vi "CRYO_MASTER_temp.vi"() -> ()   [LabVIEW 2017] (continued)
  out "LastMeasurementConfig (336)":T10(array[cluster])=[{"LSIName"="LSi336X", "Active?"=TRUE, "LastData"=[295.892, 295.621, 295.543, 295.514], "Labels"=["T1K3-1", "T1K3-2", "T3He5", "T3He8"]}, {"LSIName"="LSi336Y", "Active?"=TRUE, "LastData"=[295.418, 295.377, 295.467, 295.916], "Labels"=["T3He6-1", "T3He6-2", "T3He7-1", "T3He7-2"]}]
  out "DataArrayConv (USB) 2":dbl[][](array[numeric])
  # "GLOBAL STATUS/CONTROL"
  # "USB6210 Analog inputs Settings"
  # "USB6218 Analog inputs Settings"
  # "USB6218 Dewar Pressure Regulation"
  # "Global Settings"
  # "LSI218 Settings"
  # "LSI336 Settings"
  # "LSI218 Settings"
  # "Graph screenshots"
  # "Configuration"
  # "Vavle Status"
  # "OPEN"
  # "CLOSED"
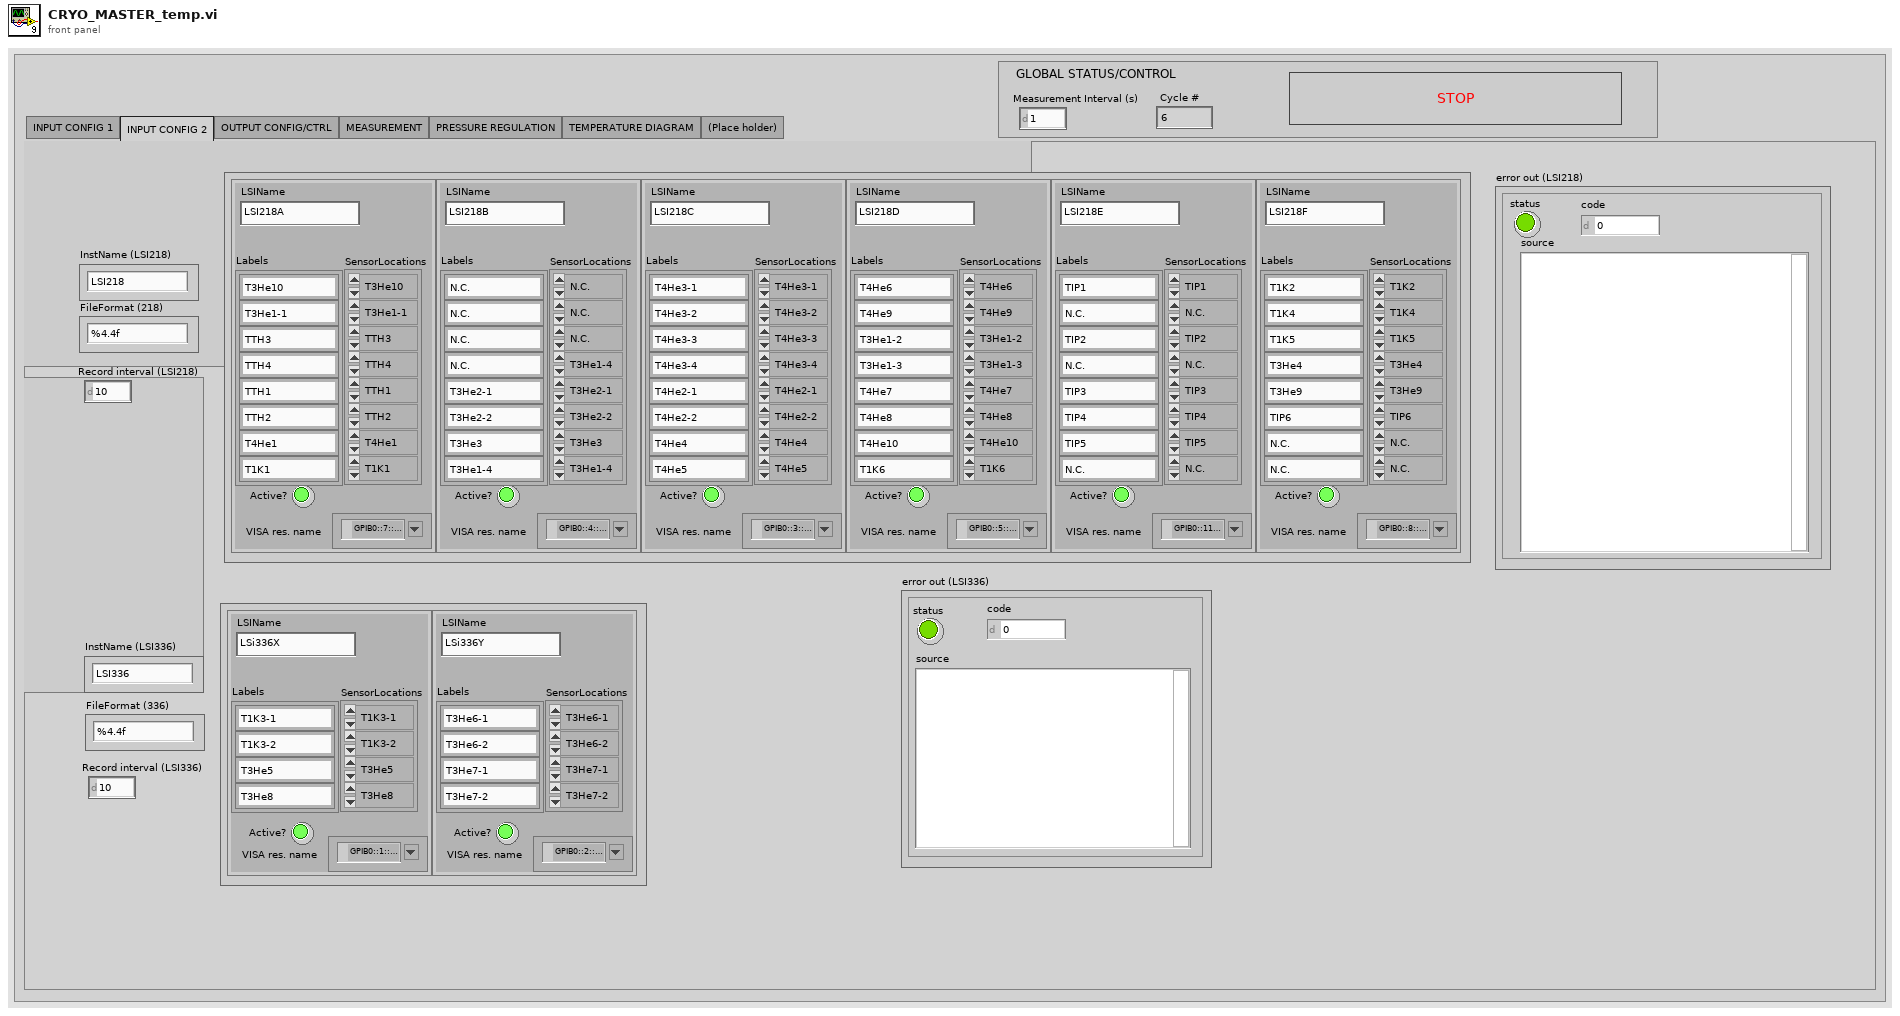
[diagram p1: front panel]
types:
  T1 = enum32{"INPUT CONFIG 1", "INPUT CONFIG 2", "OUTPUT CONFIG/CTRL", "MEASUREMENT", "PRESSURE REGULATION", "TEMPERATURE DIAGRAM", "(Place holder)"}
  T2 = cluster{"Label":string, "FileFormat":string, "Active?":bool, "Physical CH":tag, " terminal\n type":i32, "ConversionType":cluster{"Type":enum16{"Raw", "SimpleProp", "CC-10_COMBINED", "CC-10_LOG", "LeakDet_EXP", "LeakDet_Mantissa", "Baratron"}, "ConversionParameters":dbl[]}, "VoltageLimits":dbl[]}[]
  T3 = cluster{"LSIName":string, "Labels":string[], "SensorLocations":enum16{"N.C.", "T3He1-1", "T3He1-2", "T3He1-3", "T3He1-4", "T3He2-1", "T3He2-2", "T3He3", "T3He4", "T3He5", "T3He6-1", "T3He6-2", "T3He7-1", "T3He7-2", "T3He8", "T3He9", "T3He10", "T4He1", "T4He2-1", "T4He2-2", "T4He3-1", "T4He3-2", "T4He3-3", "T4He3-4", "T4He4", "T4He5", "T4He6", "T4He7", "T4He8", "T4He9", "T4He10", "T1K1", "T1K2", "T1K3-1", "T1K3-2", "T1K4", "T1K5", "T1K6", "TIP1", "TIP2", "TIP3", "TIP4", "TIP5", "TIP6", "TIP7", "TTH1", "TTH2", "TTH3", "TTH4"}[], "Active?":bool, "VISA res. name":refnum<visa-resource-name>}[]
  T4 = enum32{"USB6210", "USB6218", "Temeprature (1)", "Temperature (2)", "Temperature (3)"}
  T5 = enum16{"Intialized", "Ready", "Measuring", "Terminated"}
  T6 = enum16{"Initialized", "Ready", "Measuring", "Terminated"}
  T7 = cluster{"TimeArray":timestamp[], "LDArray":dbl[]}[]
  T8 = cluster{"TimeArray":timestamp[], "DataArray":dbl[]}[]
  T9 = cluster{"TimeArray":timestamp[], "Filtered X":dbl[]}[]
  T10 = cluster{"LSIName":string, "Active?":bool, "LastData":dbl[], "Labels":string[]}[]
  T11 = enum16{"Undefined", "Initialized", "Pressurizing", "Depressurizing"}
  T12 = cluster{"TimeArray":timestamp[], "DataArrayConv":dbl[]}[]
  T13 = cluster{"IndexArray":i64[], "TimeArray":timestamp[], "DataArrayRaw":dbl[][], "DataArrayConv":dbl[][], "LDArray":dbl[]}
  T14 = cluster{"InstName":string, "Active?":bool, "Status":enum16{"Intialized", "Ready", "Measuring", "Terminated"}, "Labels":string[], "LabelLD":string, "FileFormat":string[], "FileFormatLD":string, "ReadLeakDet?":bool}
  T15 = cluster{"TimeArray":timestamp[], "DataArrayConv":dbl[]}
  T16 = cluster{"TimeArray":timestamp[], "Filtered X":dbl[]}
  T17 = cluster{"TimeArray":timestamp[], "DataArray":dbl[]}
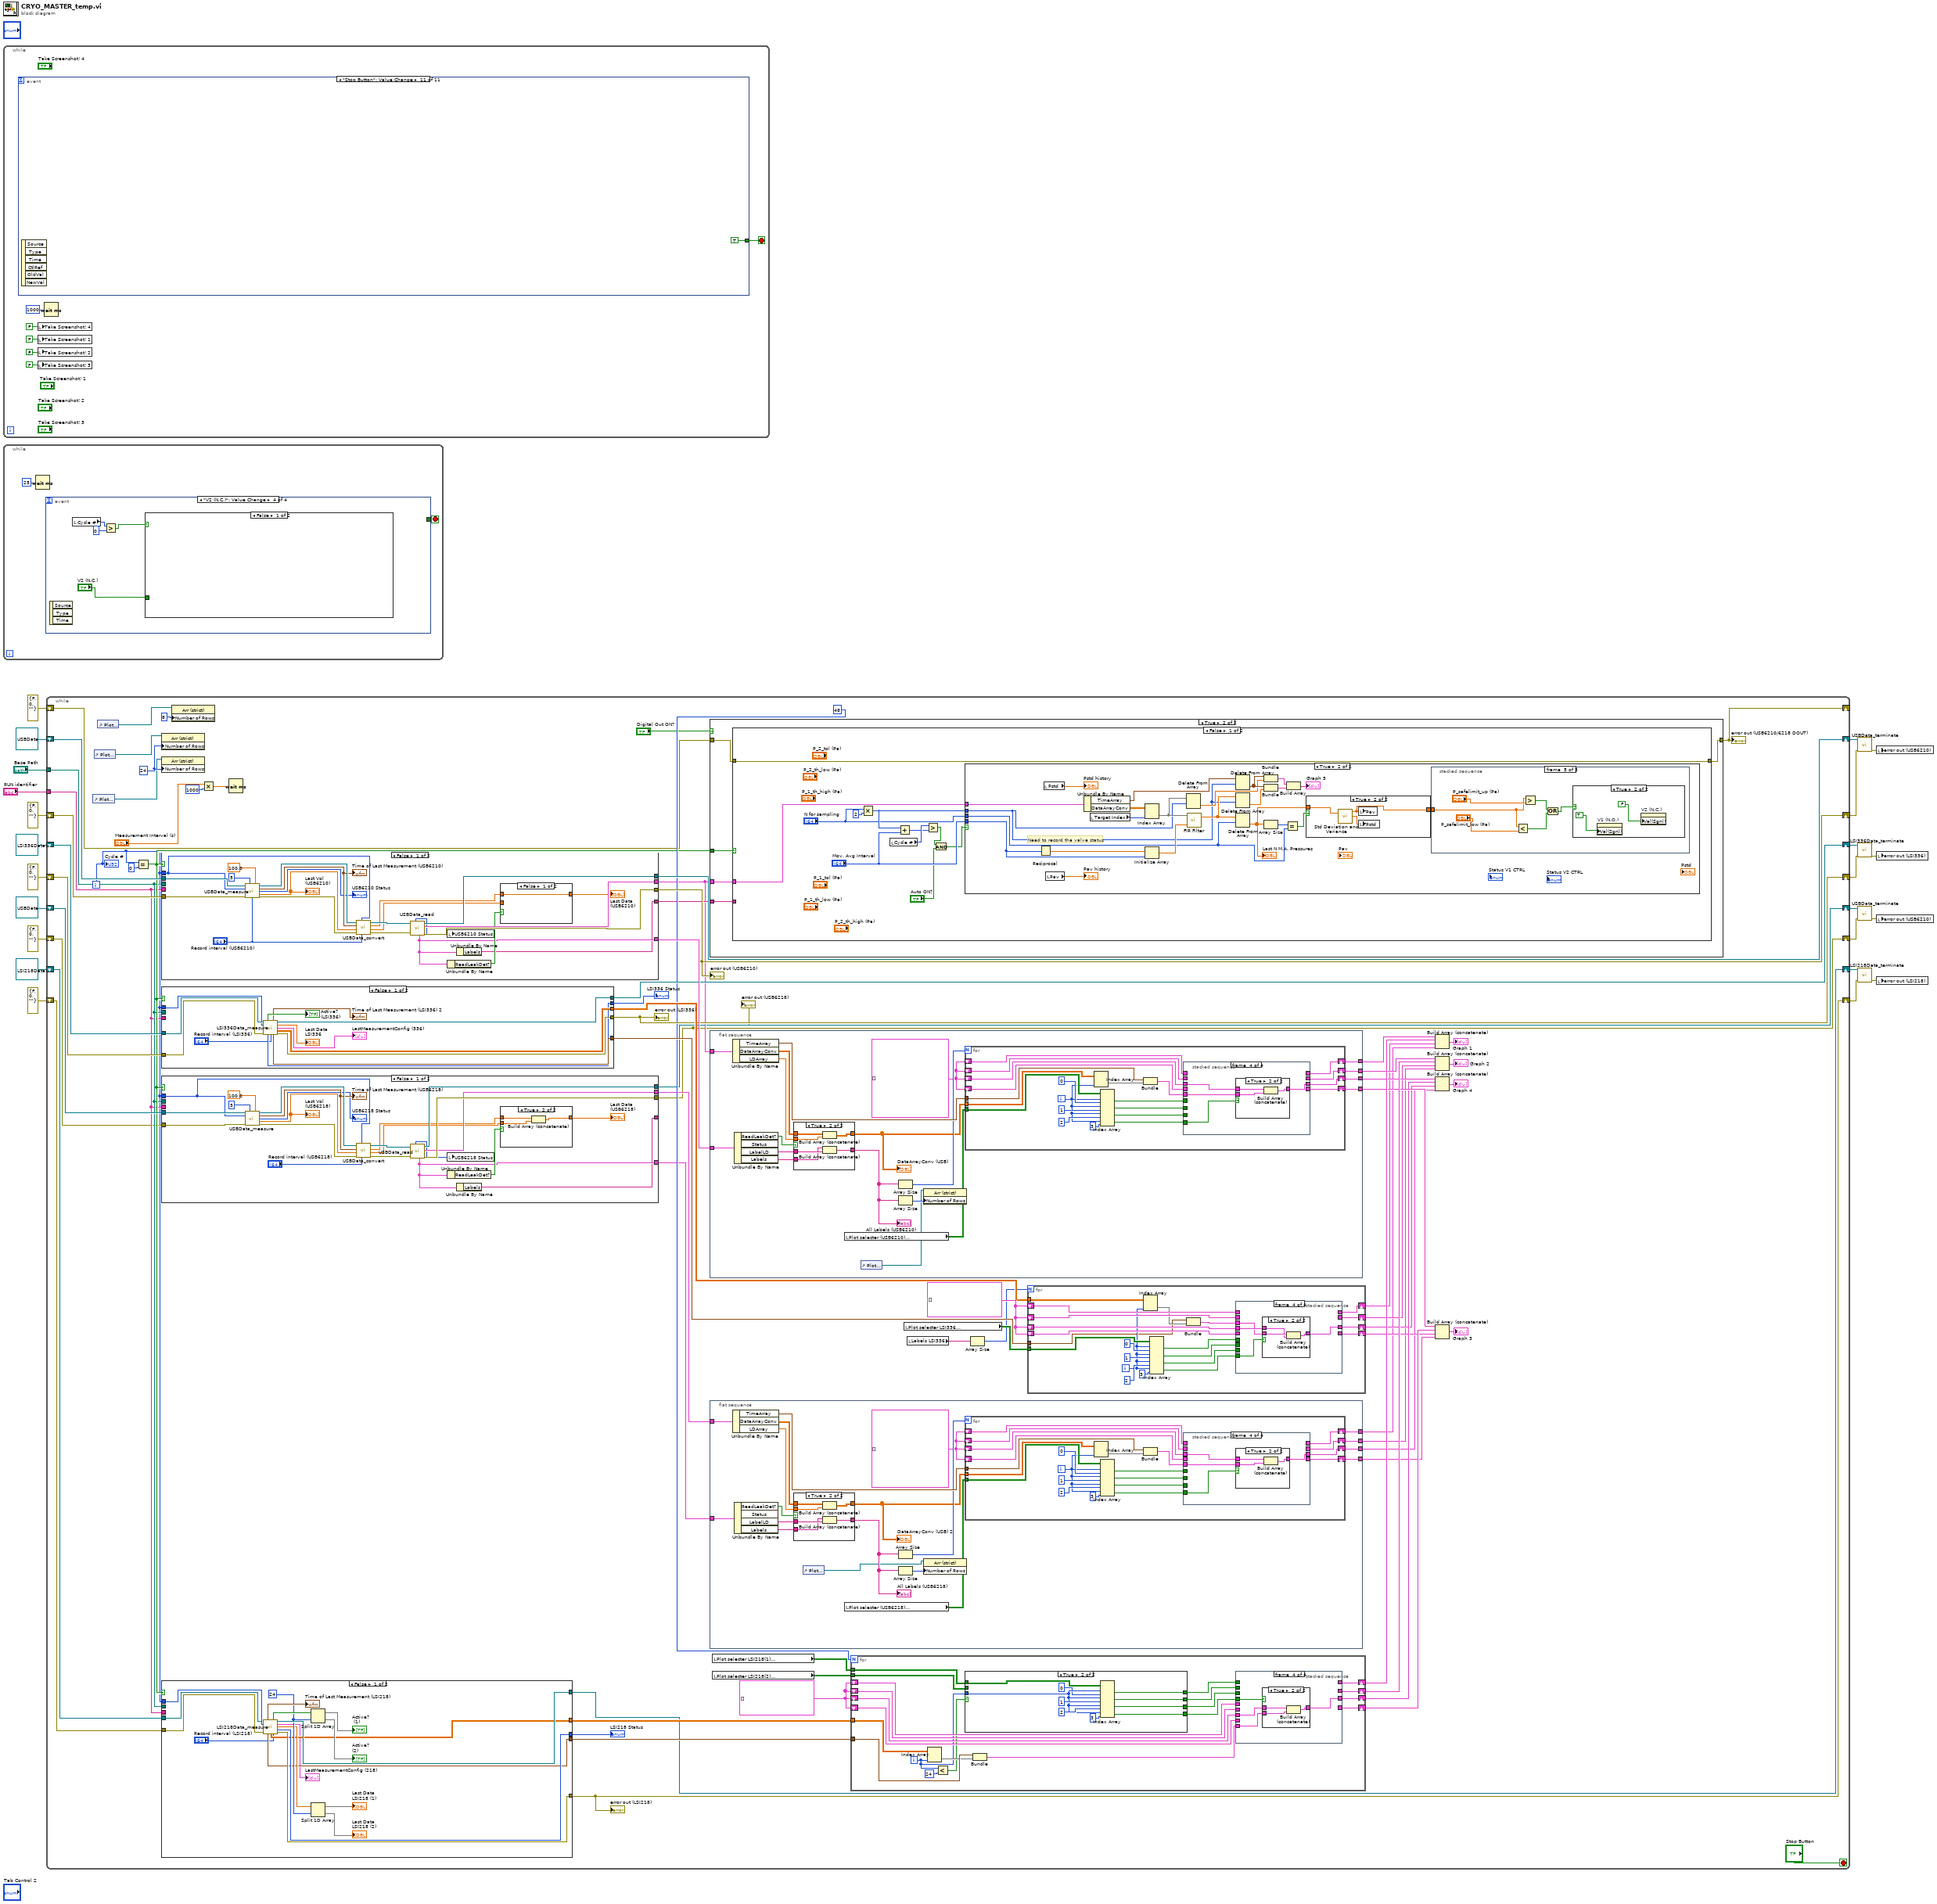
[diagram p0: block diagram]
diagram:
  n1 = while {
    stop <- w27 stop-if-true
    n2 = event shown="[10] \"Stop Button\": Value Change" {
      selector: _ -> [_ _ _ _ _ _ _ _ _ _ _]
      dyn-events: _ -> [_ _ _ _ _ _ _ _ _ _ _]
      timeout: _ -> [_ _ _ _ _ _ _ _ _ _ _]
      tunnel: [_ _ _ _ _ _ _ _ _ _ TRUE] -> w27
      event Timeout {
        n3 = event-data() -> ()  [unwired: 1 in, 3 out]
      }
      event "log/linear 1": Value Change {
        n4 = event-data() -> ()  [unwired: 1 in, 6 out]
        n5 = flat-sequence {
          frame #0 {
            n6 = control-ref of="Graph 1"() -> (w33:refnum<vi>)
            n7 = Boolean To (0,1)(Boolean="log/linear 1") -> (0, 1=w34:i16)
            n8 = property class="XYGraph (strict)"(reference=w33, error in=errorcluster {"status"=FALSE, "code"=0, "source"=""} ("error in (no error)"), "YScale.Mapping Mode"=w34) -> (error out=w31:errorcluster)  [unwired: 1 out]
            n9 = control-ref of="error out (USB6210)"() -> (w32:refnum<vi>)
            n10 = property class="Clust (strict)"(reference=w32, "Val(Sgnl)"=w31) -> ()  [unwired: 1 in, 2 out]
          }
        }
      }
      event "log/linear 2": Value Change {
        n11 = event-data() -> ()  [unwired: 1 in, 6 out]
        n12 = flat-sequence {
          frame #0 {
            n13 = control-ref of="Graph 2"() -> (w38:refnum<vi>)
            n14 = Boolean To (0,1)(Boolean="log/linear 2") -> (0, 1=w40:i16)
            n15 = property class="XYGraph (strict)"(reference=w38, error in=errorcluster {"status"=FALSE, "code"=0, "source"=""} ("error in (no error)"), "YScale.Mapping Mode"=w40) -> (error out=w39:errorcluster)  [unwired: 1 out]
            n16 = control-ref of="error out (USB6210)"() -> (w37:refnum<vi>)
            n17 = property class="Clust (strict)"(reference=w37, "Value"=w39) -> ()  [unwired: 1 in, 2 out]
          }
        }
      }
      event "log/linear 3": Value Change {
        n18 = event-data() -> ()  [unwired: 1 in, 6 out]
        n19 = flat-sequence {
          frame #0 {
            n20 = control-ref of="Graph 3"() -> (w42:refnum<vi>)
            n21 = Boolean To (0,1)(Boolean="log/linear 3") -> (0, 1=w46:i16)
            n22 = property class="XYGraph (strict)"(reference=w42, error in=errorcluster {"status"=FALSE, "code"=0, "source"=""} ("error in (no error)"), "YScale.Mapping Mode"=w46) -> (error out=w45:errorcluster)  [unwired: 1 out]
            n23 = control-ref of="error out (USB6210)"() -> (w44:refnum<vi>)
            n24 = property class="Clust (strict)"(reference=w44, "Value"=w45) -> ()  [unwired: 1 in, 2 out]
          }
        }
      }
      event "log/linear 4": Value Change {
        n25 = event-data() -> ()  [unwired: 1 in, 6 out]
        n26 = flat-sequence {
          frame #0 {
            n27 = control-ref of="Graph 4"() -> (w48:refnum<vi>)
            n28 = Boolean To (0,1)(Boolean="log/linear 4") -> (0, 1=w52:i16)
            n29 = property class="XYGraph (strict)"(reference=w48, error in=errorcluster {"status"=FALSE, "code"=0, "source"=""} ("error in (no error)"), "YScale.Mapping Mode"=w52) -> (error out=w51:errorcluster)  [unwired: 1 out]
            n30 = control-ref of="error out (USB6210)"() -> (w50:refnum<vi>)
            n31 = property class="Clust (strict)"(reference=w50, "Value"=w51) -> ()  [unwired: 1 in, 2 out]
          }
        }
      }
      event "Plot selecter LSI218(1)\n    1      2     3     4", "Plot selecter LSI218(2)\n    1      2     3     4", "Plot selecter (USB6210)\n    1      2     3     4", "Plot selecter LSI336 \n     1      2     3     4", "Plot selecter (USB6218)\n    1      2     3     5": Value Change {
        n32 = event-data() -> ()  [unwired: 1 in, 6 out]
        n33 = local read "All Labels (USB6210)"() -> (w70:string[])
        n34 = local read "All Labels (USB6218)"() -> (w59:string[])
        n35 = local read "Labels LSI218 (1)"() -> (w72:string[])
        n36 = local read "Labels LSI218 (2)"() -> (w73:string[])
        n37 = local read "Labels LSI336"() -> (w65:string[])
        n38 = call "BuildPlotLegends.vi"("Plot selecter \n    1      2     3     4"="Plot selecter (USB6210)\n    1      2     3     4", "AllLabels"=w70) -> ("Series 4"=w82:string[], "Series 3"=w80:string[], "Series 2"=w78:string[], "Series 1"=w76:string[])  [unwired: 6 in]
        n39 = call "BuildPlotLegends_LSI218.vi"("Plot selecter (2)\n    1      2     3     5"="Plot selecter LSI218(2)\n    1      2     3     4", "Plot selecter (1)\n    1      2     3     4"="Plot selecter LSI218(1)\n    1      2     3     4", "Labels (2)"=w73, "Labels (1)"=w72) -> ("Series 4"=w83:string[], "Series 3"=w81:string[], "Series 2"=w79:string[], "Series 1"=w77:string[])  [unwired: 4 in]
        n40 = call "BuildPlotLegends.vi"("Plot selecter \n    1      2     3     4"="Plot selecter LSI336 \n     1      2     3     4", "AllLabels"=w65) -> ("Series 4"=w60:string[], "Series 3"=w61:string[], "Series 2"=w62:string[], "Series 1"=w63:string[])  [unwired: 6 in]
        n41 = call "BuildPlotLegends.vi"("Plot selecter \n    1      2     3     4"="Plot selecter (USB6218)\n    1      2     3     5", "AllLabels"=w59) -> ("Series 4"=w55:string[], "Series 3"=w54:string[], "Series 2"=w56:string[], "Series 1"=w57:string[])  [unwired: 6 in]
        n42 = Build Array (concatenate)(w78, w79, w62, w56) -> (w67:string[])
        "Series 2" <- w67
        n43 = Build Array (concatenate)(w80, w81, w61, w54) -> (w68:string[])
        "Series 3" <- w68
        n44 = Build Array (concatenate)(w82, w83, w60, w55) -> (w69:string[])
        "Series 4" <- w69
        n45 = Build Array (concatenate)(w76, w77, w63, w57) -> (w66:string[])
        "Series 1" <- w66
        n46 = stacked-sequence {
          tunnel: [w92 _ _ _] -> w87
          tunnel: [_ w111 _ _] -> w88
          tunnel: [_ _ w127 _] -> w86
          tunnel: [_ _ _ w144] -> w85
          tunnel: w66 -> [w89 _ _ _]
          tunnel: w67 -> [_ w107 _ _]
          tunnel: w68 -> [_ _ w124 _]
          tunnel: w69 -> [_ _ _ w141]
          frame #0 {
            n47 = Array Size(array=w89) -> (size(s)=w95:i32)
            n48 = control-ref of="Graph 1"() -> (w93:refnum<vi>)
            n49 = for {
              N: 18 -> [_]
              tunnel: w93 -> [w104]
              shift-right: [w102] -> w94
              shift-left: errorcluster {"status"=FALSE, "code"=0, "source"=""} ("error in (no error)") -> [w103]
              i -> [w106]
              n50 = property class="XYGraph (strict)"(reference=w104, error in=w103, "Active Plot"=w106, "Plot.Plot Name"="") -> (error out=w102:errorcluster)  [unwired: 1 out]
            }
            n51 = for {
              N: w95 -> [_]
              tunnel: w93 -> [w100]
              shift-right: [w98] -> w92
              shift-left: w94 -> [w99]
              tunnel: w89 -> [w97] mode=indexing
              i -> [w101]
              n52 = property class="XYGraph (strict)"(reference=w100, error in=w99, "Active Plot"=w101, "Plot.Plot Name"=w97, "Plot.Visible?"=TRUE ("Plot.Visible")) -> (error out=w98:errorcluster)  [unwired: 1 out]
            }
          }
          frame #1 {
            n53 = Array Size(array=w107) -> (size(s)=w113:i32)
            n54 = control-ref of="Graph 2"() -> (w110:refnum<vi>)
            n55 = for {
              N: 18 -> [_]
              shift-right: [w120] -> w112
              shift-left: errorcluster {"status"=FALSE, "code"=0, "source"=""} ("error in (no error)") -> [w121]
              tunnel: w110 -> [w119]
              i -> [w123]
              n56 = property class="XYGraph (strict)"(reference=w119, error in=w121, "Active Plot"=w123, "Plot.Plot Name"="") -> (error out=w120:errorcluster)  [unwired: 1 out]
            }
            n57 = for {
              N: w113 -> [_]
              shift-right: [w116] -> w111
              shift-left: w112 -> [w117]
              tunnel: w107 -> [w115] mode=indexing
              tunnel: w110 -> [w114]
              i -> [w118]
              n58 = property class="XYGraph (strict)"(reference=w114, error in=w117, "Active Plot"=w118, "Plot.Plot Name"=w115) -> (error out=w116:errorcluster)  [unwired: 1 out]
            }
          }
          frame #2 {
            n59 = Array Size(array=w124) -> (size(s)=w130:i32)
            n60 = control-ref of="Graph 3"() -> (w128:refnum<vi>)
            n61 = for {
              N: 18 -> [_]
              tunnel: w128 -> [w138]
              shift-right: [w136] -> w129
              shift-left: errorcluster {"status"=FALSE, "code"=0, "source"=""} ("error in (no error)") -> [w137]
              i -> [w140]
              n62 = property class="XYGraph (strict)"(reference=w138, error in=w137, "Active Plot"=w140, "Plot.Plot Name"="") -> (error out=w136:errorcluster)  [unwired: 1 out]
            }
            n63 = for {
              N: w130 -> [_]
              tunnel: w128 -> [w134]
              shift-right: [w132] -> w127
              shift-left: w129 -> [w133]
              tunnel: w124 -> [w131] mode=indexing
              i -> [w135]
              n64 = property class="XYGraph (strict)"(reference=w134, error in=w133, "Active Plot"=w135, "Plot.Plot Name"=w131) -> (error out=w132:errorcluster)  [unwired: 1 out]
            }
          }
          frame #3 {
            n65 = Array Size(array=w141) -> (size(s)=w147:i32)
            n66 = control-ref of="Graph 4"() -> (w145:refnum<vi>)
            n67 = for {
              N: 18 -> [_]
              tunnel: w145 -> [w155]
              shift-right: [w153] -> w146
              shift-left: errorcluster {"status"=FALSE, "code"=0, "source"=""} ("error in (no error)") -> [w154]
              i -> [w157]
              n68 = property class="XYGraph (strict)"(reference=w155, error in=w154, "Active Plot"=w157, "Plot.Plot Name"="") -> (error out=w153:errorcluster)  [unwired: 1 out]
            }
            n69 = for {
              N: w147 -> [_]
              tunnel: w145 -> [w151]
              shift-right: [w149] -> w144
              shift-left: w146 -> [w150]
              tunnel: w141 -> [w148] mode=indexing
              i -> [w152]
              n70 = property class="XYGraph (strict)"(reference=w151, error in=w150, "Active Plot"=w152, "Plot.Plot Name"=w148) -> (error out=w149:errorcluster)  [unwired: 1 out]
            }
          }
        }
        n71 = Merge Errors(w87, w88, w86, w85) -> (→"Plot errors":errorcluster)
      }
      event "Take Screenshot! 1": Value Change {
        n72 = event-data() -> ()  [unwired: 1 in, 6 out]
        n73 = flat-sequence {
          frame #0 {
            n74 = flat-sequence {
              frame #0 {
                w161 = "_" ("string")
                n75 = Get Date/Time In Seconds() -> (seconds since 1Jan1904=w158:timestamp)
                n76 = local read "RUN identifier"() -> (w165:string)
                n77 = call "LV_UNIXTIME.vi"("current time"=w158) -> ("date/time string"=w162:string)  [unwired: 9 in, 1 out]
                n78 = local read "Base Path"() -> (w166:path)
                n79 = Concatenate Strings(w165, w161, w162, w161, "FIle suffix 1", ".bmp" ("string")) -> (w171:string)
                n80 = control-ref of="Graph 1"() -> (w163:refnum<vi>)
                n81 = Build Path(base path=w166, name or relative path=w171) -> (appended path=w170:path)
                n82 = invoke on="Invoke Node" class="XYGraph (strict)" method="Export Image"(reference=w163, "FileType"=enum32{"BMP", "EPS", "EMF", "PICT"}."BMP" ("File Type"), "Target"=enum32{"File", "Clipboard"}."File", "Path"=w170, "HideGrid"=FALSE ("Hide Grid"), "Overwrite"=TRUE ("Always Overwrite")) -> ()  [unwired: 2 in, 8 out]
              }
              frame #1 {
                n83 = local write "Take Screenshot! 1"(FALSE ("Take Screenshot! 1")) -> ()
              }
            }
          }
        }
      }
      event "Take Screenshot! 2": Value Change {
        n84 = event-data() -> ()  [unwired: 1 in, 6 out]
        n85 = flat-sequence {
          frame #0 {
            n86 = flat-sequence {
              frame #0 {
                w177 = "_" ("string")
                n87 = Get Date/Time In Seconds() -> (seconds since 1Jan1904=w173:timestamp)
                n88 = local read "RUN identifier"() -> (w180:string)
                n89 = call "LV_UNIXTIME.vi"("current time"=w173) -> ("date/time string"=w178:string)  [unwired: 9 in, 1 out]
                n90 = local read "Base Path"() -> (w181:path)
                n91 = Concatenate Strings(w180, w177, w178, w177, "FIle suffix 2", ".bmp" ("string")) -> (w186:string)
                n92 = control-ref of="Graph 2"() -> (w174:refnum<vi>)
                n93 = Build Path(base path=w181, name or relative path=w186) -> (appended path=w185:path)
                n94 = invoke on="Invoke Node" class="XYGraph (strict)" method="Export Image"(reference=w174, "FileType"=enum32{"BMP", "EPS", "EMF", "PICT"}."BMP" ("File Type"), "Target"=enum32{"File", "Clipboard"}."File", "Path"=w185, "HideGrid"=FALSE ("Hide Grid"), "Overwrite"=TRUE ("Always Overwrite")) -> ()  [unwired: 2 in, 8 out]
              }
              frame #1 {
                n95 = local write "Take Screenshot! 2"(FALSE ("Take Screenshot! 1")) -> ()
              }
            }
          }
        }
      }
      event "Take Screenshot! 3": Value Change {
        n96 = event-data() -> ()  [unwired: 1 in, 6 out]
        n97 = flat-sequence {
          frame #0 {
            n98 = flat-sequence {
              frame #0 {
                w192 = "_" ("string")
                n99 = Get Date/Time In Seconds() -> (seconds since 1Jan1904=w190:timestamp)
                n100 = local read "RUN identifier"() -> (w195:string)
                n101 = call "LV_UNIXTIME.vi"("current time"=w190) -> ("date/time string"=w193:string)  [unwired: 9 in, 1 out]
                n102 = local read "Base Path"() -> (w196:path)
                n103 = Concatenate Strings(w195, w192, w193, w192, "FIle suffix 3", ".bmp" ("string")) -> (w201:string)
                n104 = control-ref of="Graph 3"() -> (w188:refnum<vi>)
                n105 = Build Path(base path=w196, name or relative path=w201) -> (appended path=w200:path)
                n106 = invoke on="Invoke Node" class="XYGraph (strict)" method="Export Image"(reference=w188, "FileType"=enum32{"BMP", "EPS", "EMF", "PICT"}."BMP" ("File Type"), "Target"=enum32{"File", "Clipboard"}."File", "Path"=w200, "HideGrid"=FALSE ("Hide Grid"), "Overwrite"=TRUE ("Always Overwrite")) -> ()  [unwired: 2 in, 8 out]
              }
              frame #1 {
                n107 = local write "Take Screenshot! 3"(FALSE ("Take Screenshot! 1")) -> ()
              }
            }
          }
        }
      }
      event "Take Screenshot! 4": Value Change {
        n108 = event-data() -> ()  [unwired: 1 in, 6 out]
        n109 = flat-sequence {
          frame #0 {
            n110 = flat-sequence {
              frame #0 {
                w207 = "_" ("string")
                n111 = Get Date/Time In Seconds() -> (seconds since 1Jan1904=w205:timestamp)
                n112 = local read "RUN identifier"() -> (w210:string)
                n113 = call "LV_UNIXTIME.vi"("current time"=w205) -> ("date/time string"=w208:string)  [unwired: 9 in, 1 out]
                n114 = local read "Base Path"() -> (w211:path)
                n115 = Concatenate Strings(w210, w207, w208, w207, "FIle suffix 4", ".bmp" ("string")) -> (w216:string)
                n116 = control-ref of="Graph 4"() -> (w203:refnum<vi>)
                n117 = Build Path(base path=w211, name or relative path=w216) -> (appended path=w215:path)
                n118 = invoke on="Invoke Node" class="XYGraph (strict)" method="Export Image"(reference=w203, "FileType"=enum32{"BMP", "EPS", "EMF", "PICT"}."BMP" ("File Type"), "Target"=enum32{"File", "Clipboard"}."File", "Path"=w215, "HideGrid"=FALSE ("Hide Grid"), "Overwrite"=TRUE ("Always Overwrite")) -> ()  [unwired: 2 in, 8 out]
              }
              frame #1 {
                n119 = local write "Take Screenshot! 4"(FALSE ("Take Screenshot! 1")) -> ()
              }
            }
          }
        }
      }
      event "Stop Button": Value Change {
        n120 = event-data() -> ()  [unwired: 1 in, 6 out]
      }
    }
    n121 = local write "Take Screenshot! 4"(FALSE ("Take Screenshot! 1")) -> ()
    n122 = local write "Take Screenshot! 1"(FALSE ("Take Screenshot! 1")) -> ()
    n123 = local write "Take Screenshot! 2"(FALSE ("Take Screenshot! 1")) -> ()
    n124 = local write "Take Screenshot! 3"(FALSE ("Take Screenshot! 1")) -> ()
    n125 = Wait (ms)(milliseconds to wait=u32 1000) -> ()  [unwired: 1 out]
  }
  n126 = while {
    stop <- w219 stop-if-true
    n127 = Wait (ms)(milliseconds to wait=u32 25) -> ()  [unwired: 1 out]
    n128 = event shown="[3] \"V2 (N.C.)\": Value Change" {
      selector: _ -> [_ _ _ _]
      dyn-events: _ -> [_ _ _ _]
      timeout: _ -> [_ _ _ _]
      tunnel: [_ TRUE _ _] -> w219
      event Timeout {
        n129 = event-data() -> ()  [unwired: 1 in, 3 out]
      }
      event "Stop Button": Value Change {
        n130 = event-data() -> ()  [unwired: 1 in, 3 out]
        n131 = local read "DOUT task out"() -> (w222:refnum<k21>)
        n132 = call <vilib>:"DAQmx Clear Task.vi"("task in"=w222, "error in"=errorcluster {"status"=FALSE, "code"=0, "source"=""}) -> ("error out"=w223:errorcluster)  [unwired: 13 in]
        n133 = local write "error out (USB6210/6218 DOUT)"(w223) -> ()
      }
      event "V1 (N.O.)": Value Change {
        n134 = event-data() -> ()  [unwired: 1 in, 3 out]
        n135 = local read "Cycle #"() -> (w227:u32)
        n136 = Greater?(x=w227, y=u32 0) -> (0:w225:bool)
        n137 = case shown="True" w225 {
          tunnel: "V1 (N.O.)" -> [_ w234]
          tunnel: "V1 (N.O.)" -> [_ w230]
          frame False {
          }
          frame True {
            n138 = Not(x=w230) -> (.not. x?=w235:bool)
            n139 = case shown="True" w234 {
              frame False {
                (unwired) T11."Pressurizing" ("V1 Status")
              }
              frame True {
                (unwired) T11."Depressurizing" ("V1 Status")
              }
            }
            n140 = property on="V2 (N.C.)" class="Bool (strict)"() -> ("Value"=w229:bool)  [unwired: 2 in, 2 out]
            n141 = local read "error out (USB6210/6218 DOUT)"() -> (w232:errorcluster)
            n142 = local read "DOUT task out"() -> (w238:refnum<k21>)
            n143 = Build Array(w235, w229) -> (w233:bool[])
            n144 = call <vilib>:"DAQmx Write (Digital 1D Bool NChan 1Samp 1Line).vi"("task/channels in"=w238, "data"=w233, "timeout"=10.0, "error in"=w232) -> ("task out"=w236:refnum<k21>, "error out"=w231:errorcluster)  [unwired: 9 in, 1 out]
            n145 = local write "DOUT task out"(w236) -> ()
            n146 = local write "error out (USB6210/6218 DOUT)"(w231) -> ()
          }
        }
      }
      event "V2 (N.C.)": Value Change {
        n147 = event-data() -> ()  [unwired: 1 in, 3 out]
        n148 = local read "Cycle #"() -> (w241:u32)
        n149 = Greater?(x=w241, y=u32 0) -> (0:w239:bool)
        n150 = case shown="False" w239 {
          tunnel: "V2 (N.C.)" -> [_ w246]
          frame False {
          }
          frame True {
            n151 = case shown="True" w246 {
              frame False {
                (unwired) T11."Pressurizing" ("V1 Status")
              }
              frame True {
                (unwired) T11."Depressurizing" ("V1 Status")
              }
            }
            n152 = local read "error out (USB6210/6218 DOUT)"() -> (w250:errorcluster)
            n153 = property on="V1 (N.O.)" class="Bool (strict)"() -> ("Value"=w244:bool)  [unwired: 2 in, 2 out]
            n154 = Not(x=w244) -> (.not. x?=w243:bool)
            n155 = local read "DOUT task out"() -> (w251:refnum<k21>)
            n156 = Build Array(w243, w246) -> (w247:bool[])
            n157 = call <vilib>:"DAQmx Write (Digital 1D Bool NChan 1Samp 1Line).vi"("task/channels in"=w251, "data"=w247, "timeout"=10.0, "error in"=w250) -> ("task out"=w248:refnum<k21>, "error out"=w245:errorcluster)  [unwired: 9 in, 1 out]
            n158 = local write "DOUT task out"(w248) -> ()
            n159 = local write "error out (USB6210/6218 DOUT)"(w245) -> ()
          }
        }
      }
    }
  }
  n160 = while {
    shift-right: [w318] -> w20
    shift-left: refnum<class "USBData.lvclass"> refnum ("USBData.lvclass") -> [w322]
    shift-right: [w314] -> w19
    shift-left: errorcluster {"status"=FALSE, "code"=0, "source"=""} ("error in (no error)") -> [w321]
    tunnel: "RUN identifier" -> [w262]
    tunnel: "Base Path" -> [w263]
    shift-right: [w294] -> w13
    shift-left: errorcluster {"status"=FALSE, "code"=0, "source"=""} ("error in (no error)") -> [w312]
    shift-right: [w295] -> w14
    shift-left: refnum<class "LSI218Data.lvclass"> refnum ("LSI218Data.lvclass") -> [w311]
    shift-right: [w280] -> w9
    shift-left: refnum<class "LSI336Data.lvclass"> refnum ("LSI336Data.lvclass") -> [w291]
    shift-right: [w279] -> w8
    shift-left: errorcluster {"status"=FALSE, "code"=0, "source"=""} ("error in (no error)") -> [w290]
    shift-right: [w267] -> _
    shift-left: errorcluster {"status"=FALSE, "code"=0, "source"=""} ("error in") -> [w268]
    shift-right: [w253] -> w2
    shift-left: refnum<class "USBData.lvclass"> refnum ("USBData.lvclass") -> [w265]
    shift-right: [w252] -> w1
    shift-left: errorcluster {"status"=FALSE, "code"=0, "source"=""} ("error in (no error)") -> [w261]
    i -> [w260]
    stop <- "Stop Button" stop-if-true
    w275 = u32 24 ("Number of Rows")
    w287 = T12 [] ("appended array")
    w305 = T12 [] ("appended array")
    n161 = control-ref of="Plot selecter LSI218(2)\n    1      2     3     4"() -> (w273:refnum<vi>)
    n162 = control-ref of="Plot selecter LSI218(1)\n    1      2     3     4"() -> (w274:refnum<vi>)
    n163 = control-ref of="Plot selecter LSI336 \n     1      2     3     4"() -> (w272:refnum<vi>)
    n164 = Equal?(x=w260, y=0) -> (x = y?=w264:bool)
    n165 = property on="Property Node" class="Arr (strict)"(reference=w274, "Number of Rows"=w275) -> ()  [unwired: 1 in, 2 out]
    n166 = property on="Property Node" class="Arr (strict)"(reference=w273, "Number of Rows"=w275) -> ()  [unwired: 1 in, 2 out]
    n167 = case shown="False" w264 {
      tunnel: w322 -> [w879 w903]
      tunnel: w321 -> [w873 w901]
      tunnel: w260 -> [w864 _]
      tunnel: [w871 w898] -> w314
      tunnel: [w868 w897] -> w266
      tunnel: [w869 w896] -> w318
      tunnel: [w859 w891] -> w319
      tunnel: w262 -> [_ w889]
      tunnel: w263 -> [_ w888]
      tunnel: [w858 w885] -> w269
      frame False {
        n168 = call-dynamic "USBData_measure.vi"("USBData in"=w879, "DAQ sample #"=i64 5, "DAQ timeout"=100.0 ("DAQ timeout (def: 100)"), "MeasurementIndex"=w864, "error in (no error)"=w873, "save every ... measurements"="Record interval (USB6210)") -> ("USBData out"=w878:refnum<class "USBData.lvclass">, "TimeMeasuremeent"=w875:timestamp, "Status"=→"USB6210 Status":T5, "LastDataAcquired"=w860:dbl[], "error out"=w874:errorcluster)  [unwired: 3 in, 2 out]
        "Time of Last Measurement (USB6210)" <- w875
        "Last Vol\n(USB6210)" <- w860
        n169 = call-dynamic "USBData_convert.vi"("Save every ... measurements"="Record interval (USB6210)", "MeasurementIndex"=w864, "error in (no error)"=w874, "LastDataAcquired"=w860, "TimeMeasuremeent"=w875, "USBData in"=w878) -> ("error out"=w872:errorcluster, "LeakDet_FULL"=w867:dbl, "LastDataConverted"=w861:dbl[], "USBData out"=w870:refnum<class "USBData.lvclass">)  [unwired: 2 in]
        n170 = call "USBData_read.vi"("USBData in"=w870, "error in (no error)"=w872) -> ("Status"=w862:T5, "USBData out"=w869:refnum<class "USBData.lvclass">, "Data"=w868:T13, "Basic"=w859:T14, "error out"=w871:errorcluster)  [unwired: 2 in, 2 out]
        n171 = local write "USB6210 Status"(w862) -> ()
        n172 = Unbundle By Name(w859) -> ("ReadLeakDet?"=w866:bool)
        n173 = Unbundle By Name(w859) -> ("Labels"=w858:string[])
        n174 = case shown="False" w866 {
          tunnel: w861 -> [w880 w883]
          tunnel: w867 -> [_ w882]
          tunnel: [w880 w881] -> w865
          frame False {
          }
          frame True {
            n175 = Build Array (concatenate)(w883, w882) -> (w881:dbl[])
          }
        }
        "Last Data \n(USB6210)" <- w865
      }
      frame True {
        n176 = Get Date/Time In Seconds() -> (seconds since 1Jan1904=w890:timestamp)
        n177 = call-dynamic "USBData_initialize.vi"("USBData in"=w903, "SeriesSetting"="USB6210 Config", "BasePath"=w888, "RunName"=w889, "FileName"="InstName (USB6210)", "error in (no error)"=w901, "RUN start time"=w890) -> ("Status"=w884:T5, "USBData out"=w899:refnum<class "USBData.lvclass">, "error out"=w900:errorcluster)  [unwired: 4 in, 2 out]
        n178 = local write "USB6210 Status"(w884) -> ()
        n179 = call "USBData_read.vi"("USBData in"=w899, "error in (no error)"=w900) -> ("Status"=w887:T5, "USBData out"=w896:refnum<class "USBData.lvclass">, "Data"=w897:T13, "Basic"=w891:T14, "error out"=w898:errorcluster)  [unwired: 2 in, 2 out]
        n180 = local write "USB6210 Status"(w887) -> ()
        n181 = Unbundle By Name(w891) -> ("ReadLeakDet?"=w895:bool, "Labels"=w885:string[])
        n182 = Array Size(array=w885) -> (size(s)=w894:i32)
        n183 = case shown="True" w895 {
          tunnel: w894 -> [w904 w906]
          tunnel: [w904 w905] -> w892
          frame False {
          }
          frame True {
            n184 = Add(x=w906, y=1) -> (x+y=w905:i32)
          }
        }
        n185 = Initialize Array(TRUE ("Activate 2"), w892) -> ()  [unwired: 1 out]
      }
    }
    "error out (USB6210)" <- w314
    n186 = case shown="False" w264 {
      tunnel: [w732 w744] -> w279
      tunnel: [w722 w743] -> w289
      tunnel: [w731 w742] -> w280
      tunnel: [w730 timestamp[] [] ("TimeArray")] -> w285
      tunnel: [w729 dbl[][] [] ("DataArray")] -> w286
      tunnel: w291 -> [w728 w739]
      tunnel: w290 -> [w727 w738]
      tunnel: w262 -> [_ w736]
      tunnel: w260 -> [w723 _]
      tunnel: w263 -> [_ w733]
      frame False {
        n187 = call-dynamic "LSI336Data_measure.vi"("LSI336Data in"=w728, "MeasurementIndex"=w723, "error in (no error)"=w727, "save every ... measurements"="Record interval (LSI336)") -> ("Active?"=→"Active?\n(LSI336)":bool[], "TimeMeasuremeent"=→"Time of Last Measurement (LSI336) 2":timestamp, "LSI336Data out"=w731:refnum<class "LSI336Data.lvclass">, "LastData"=→"Last Data \nLSI336":dbl[], "LastMeasurementConfig"=→"LastMeasurementConfig (336)":T10, "DataArray"=w729:dbl[][], "Status"=w722:u16, "TimeArray"=w730:timestamp[], "error out"=w732:errorcluster)  [unwired: 3 in]
      }
      frame True {
        n188 = Get Date/Time In Seconds() -> (seconds since 1Jan1904=w745:timestamp)
        n189 = call-dynamic "LSI336Data_initialize.vi"("LSI336Data in"=w739, "RunName"=w736, "InstName"="InstName (LSI336)", "FileFormat"="FileFormat (336)", "LSI336Settings(X, Y)"="LSI336Settings(X,Y)", "RUN start time"=w745, "error in (no error)"=w738, "base path"=w733) -> ("LSI336Data out"=w742:refnum<class "LSI336Data.lvclass">, "Status"=w743:T6, "AllLabels"=→"Labels LSI336":string[], "error out"=w744:errorcluster)  [unwired: 4 in]